vi "TLB Native Dynamic Events ver 0.26e.vi"() -> ()   [LabVIEW 2018] (continued)
                      shift-right: [w1907] -> w1904
                      shift-left: w1902 -> [w1906]
                      n658 = Enqueue Element(queue=w1906, element=w1905) -> (queue out=w1907:refnum<queue>)  [unwired: 2 in, 2 out]
                    }
                  }
                  frame True {
                    n659 = for {
                      shift-right: [w1912] -> w1910
                      shift-left: w1908 -> [w1913]
                      tunnel: string[] ["READ STEPPER VALUES", "", ""] -> [w1911] mode=indexing
                      n660 = Enqueue Element(queue=w1913, element=w1911) -> (queue out=w1912:refnum<queue>)  [unwired: 2 in, 2 out]
                    }
                  }
                }
                n661 = Or(x=w1895, y=w1891) -> (x .or. y?=w1898:bool)
                n662 = Select(t=State_Type_Definitions,_for_0.26g_versions_and_later_2."True Stop" ("Enum"), s=w1891, f=State_Type_Definitions,_for_0.26g_versions_and_later_2."Task 8K: RAISE MY SWORD" ("Enum")) -> (s? t:f=w1893:T18)
                n663 = Select(t=w1893, s=w1898, f=State_Type_Definitions,_for_0.26g_versions_and_later_2."Task 8J: CLOSE CLAW" ("Enum")) -> (s? t:f=w1897:T18)
              }
              frame "Exit" {
                n664 = for {
                  shift-right: [w1920] -> w1917
                  shift-left: w1914 -> [w1921]
                  tunnel: string[] ["STOP", "RESET ENCODERS", "RESET YAW", "ARDUINO MODE 0"] -> [w1919] mode=indexing
                  n665 = Enqueue Element(queue=w1921, element=w1919) -> (queue out=w1920:refnum<queue>)  [unwired: 2 in, 2 out]
                }
              }
            }
          }
          frame 37 {
            # ">>> yStepper command>>>"
            # ">> Manual override >>"
            n666 = Dequeue Element(queue=w1932, timeout in ms (-1)=w1931, error in (no error)=w1933) -> (element=w1930:T10)  [unwired: 3 out]
            n667 = Equal?(x=w1929, y=u8 60) -> (x = y?=w1927:bool)
            n668 = case shown="\"Start Task 1\", Default" w1930 {
              tunnel: [w1943 State_Type_Definitions,_for_0.26g_versions_and_later_2."True Stop" ("Enum")] -> w1934
              tunnel: [w1946 w1963] -> w1935
              tunnel: [State_Type_Definitions,_for_0.26g_versions_and_later_2."Idle" ("Enum") State_Type_Definitions,_for_0.26g_versions_and_later_2."Shutdown" ("Enum")] -> w1936
              tunnel: w1927 -> [w1942 _]
              tunnel: w1926 -> [w1941 _]
              tunnel: w1925 -> [w1937 w1960]
              frame "Start Task 1", Default {
                # "Stays in Task 5_A until stepper reaches desired \nheight"
                # "T: Go back to idle, F: Continue with task\""
                # ">> Manual override >>"
                n669 = case shown="True" w1942 {
                  tunnel: [w1950 w1956] -> w1946
                  tunnel: w1937 -> [w1948 w1954]
                  frame False {
                    n670 = for {
                      tunnel: string[] ["Z STEPPER CAM HEIGHT", "READ STEPPER VALUES"] ("element") -> [w1951] mode=indexing
                      shift-right: [w1953] -> w1950
                      shift-left: w1948 -> [w1952]
                      n671 = Enqueue Element(queue=w1952, element=w1951) -> (queue out=w1953:refnum<queue>)  [unwired: 2 in, 2 out]
                    }
                  }
                  frame True {
                    n672 = for {
                      shift-right: [w1958] -> w1956
                      shift-left: w1954 -> [w1959]
                      tunnel: string[] ["CAM CLOSE", "DISPOSE CAM BUFFERS", "DISPOSE PROC BUFFERS", "RESET ENCODERS"] -> [w1957] mode=indexing
                      n673 = Enqueue Element(queue=w1959, element=w1957) -> (queue out=w1958:refnum<queue>)  [unwired: 2 in, 2 out]
                    }
                  }
                }
                n674 = Or(x=w1942, y=w1941) -> (x .or. y?=w1944:bool)
                n675 = Select(t=State_Type_Definitions,_for_0.26g_versions_and_later_2."True Stop" ("Enum"), s=w1941, f=State_Type_Definitions,_for_0.26g_versions_and_later_2."True Stop" ("Enum")) -> (s? t:f=w1938:T18)
                n676 = Select(t=w1938, s=w1944, f=State_Type_Definitions,_for_0.26g_versions_and_later_2."Task 8K: RAISE MY SWORD" ("Enum")) -> (s? t:f=w1943:T18)
              }
              frame "Exit" {
                n677 = for {
                  shift-right: [w1966] -> w1963
                  shift-left: w1960 -> [w1967]
                  tunnel: string[] ["STOP", "RESET ENCODERS", "RESET YAW", "ARDUINO MODE 0"] -> [w1965] mode=indexing
                  n678 = Enqueue Element(queue=w1967, element=w1965) -> (queue out=w1966:refnum<queue>)  [unwired: 2 in, 2 out]
                }
              }
            }
          }
          frame 38 {
            # ">>> Motor control cluster >>>"
            # ">> Stepper height reeached >>"
            # ">>> yStepper command>>>"
            # ">> Manual override >>"
            n679 = Dequeue Element(queue=w1979, timeout in ms (-1)=w1974, error in (no error)=w1978) -> (element=w1982:T10)  [unwired: 3 out]
            n680 = Equal?(x=w1976, y=u8 50) -> (x = y?=w1980:bool)
            n681 = case shown="\"Start Task 1\", Default" w1982 {
              tunnel: [w1993 State_Type_Definitions,_for_0.26g_versions_and_later_2."True Stop" ("Enum")] -> w1972
              tunnel: [w1991 w2008] -> w1971
              tunnel: w1975 -> [w1990 _]
              tunnel: w1977 -> [w1984 _]
              tunnel: [State_Type_Definitions,_for_0.26g_versions_and_later_2."Idle" ("Enum") State_Type_Definitions,_for_0.26g_versions_and_later_2."Shutdown" ("Enum")] -> w1973
              tunnel: w1980 -> [w1983 _]
              frame "Start Task 1", Default {
                # ">> WIill proceed to part ii if not manual override >>"
                # ">>If ENABLE or Trigger is set to true>>"
                n682 = Or(x=w1983, y=w1984) -> (x .or. y?=w1985:bool)
                n683 = case shown="False" w1983 {
                  tunnel: [w1996 w2002] -> w1991
                  tunnel: w1990 -> [w1995 w2001]
                  frame False {
                    n684 = for {
                      shift-right: [w1998] -> w1996
                      shift-left: w1995 -> [w1999]
                      tunnel: string[] ["Z STEPPER BOX HEIGHT", "READ STEPPER VALUES"] ("element") -> [w1997] mode=indexing
                      n685 = Enqueue Element(queue=w1999, element=w1997) -> (queue out=w1998:refnum<queue>)  [unwired: 2 in, 2 out]
                    }
                  }
                  frame True {
                    n686 = for {
                      shift-right: [w2004] -> w2002
                      shift-left: w2001 -> [w2005]
                      tunnel: string[] ["READ NAVX", "RESET FLAGS", "RESET YAW", "", "", ""] -> [w2003] mode=indexing
                      n687 = Enqueue Element(queue=w2005, element=w2003) -> (queue out=w2004:refnum<queue>)  [unwired: 2 in, 2 out]
                    }
                  }
                }
                n688 = Select(t=State_Type_Definitions,_for_0.26g_versions_and_later_2."True Stop" ("Enum"), s=w1984, f=State_Type_Definitions,_for_0.26g_versions_and_later_2."Task 9B: Rotate to Angle" ("Enum")) -> (s? t:f=w1987:T18)
                n689 = Select(t=w1987, s=w1985, f=State_Type_Definitions,_for_0.26g_versions_and_later_2."Task 9A: Raise Arm" ("Enum")) -> (s? t:f=w1993:T18)
              }
              frame "Exit" {
                n690 = for {
                  shift-right: [w2011] -> w2008
                  shift-left: _ -> [w2012]
                  tunnel: string[] ["STOP", "RESET ENCODERS", "RESET YAW", ""] -> [w2010] mode=indexing
                  n691 = Enqueue Element(queue=w2012, element=w2010) -> (queue out=w2011:refnum<queue>)  [unwired: 2 in, 2 out]
                }
              }
            }
          }
          frame 39 {
            # ">>> Motor control cluster >>>"
            # ">>> yStepper command>>>"
            n692 = Dequeue Element(queue=w2026, timeout in ms (-1)=w2025, error in (no error)=w2024) -> (element=w2028:T10)  [unwired: 3 out]
            n693 = In Range and Coerce(upper limit=65.0, x=w2018, lower limit=58.0) -> (In Range?=w2015:bool)  [unwired: 1 out]
            n694 = case shown="\"Start Task 1\", Default" w2028 {
              tunnel: w2019 -> [w2031 _]
              tunnel: [w2039 State_Type_Definitions,_for_0.26g_versions_and_later_2."True Stop" ("Enum")] -> w2021
              tunnel: w2027 -> [w2037 w2055]
              tunnel: [w2036 w2054] -> w2020
              tunnel: [State_Type_Definitions,_for_0.26g_versions_and_later_2."Idle" ("Enum") State_Type_Definitions,_for_0.26g_versions_and_later_2."Shutdown" ("Enum")] -> w2022
              tunnel: w2015 -> [w2029 _]
              frame "Start Task 1", Default {
                n695 = Or(x=w2029, y=w2031) -> (x .or. y?=w2030:bool)
                n696 = case shown="False" w2029 {
                  tunnel: w2037 -> [w2042 w2048]
                  tunnel: [w2041 w2046] -> w2036
                  frame False {
                    n697 = for {
                      shift-right: [w2044] -> w2041
                      shift-left: w2042 -> [w2045]
                      tunnel: string[] ["READ NAVX", "R-CW", ""] ("element") -> [w2043] mode=indexing
                      n698 = Enqueue Element(queue=w2045, element=w2043) -> (queue out=w2044:refnum<queue>)  [unwired: 2 in, 2 out]
                    }
                  }
                  frame True {
                    n699 = for {
                      shift-right: [w2050] -> w2046
                      shift-left: w2048 -> [w2051]
                      tunnel: string[] ["STOP", "RESET ENCODERS", "RESET YAW", "", ""] -> [w2049] mode=indexing
                      n700 = Enqueue Element(queue=w2051, element=w2049) -> (queue out=w2050:refnum<queue>)  [unwired: 2 in, 2 out]
                    }
                  }
                }
                n701 = Select(t=State_Type_Definitions,_for_0.26g_versions_and_later_2."True Stop" ("Enum"), s=w2031, f=State_Type_Definitions,_for_0.26g_versions_and_later_2."Task 9C: Detect Box") -> (s? t:f=w2033:T18)
                n702 = Select(t=w2033, s=w2030, f=State_Type_Definitions,_for_0.26g_versions_and_later_2."Task 9B: Rotate to Angle" ("Enum")) -> (s? t:f=w2039:T18)
              }
              frame "Exit" {
                n703 = for {
                  shift-right: [w2058] -> w2054
                  shift-left: w2055 -> [w2059]
                  tunnel: string[] ["STOP", "RESET ENCODERS", "RESET YAW", ""] -> [w2057] mode=indexing
                  n704 = Enqueue Element(queue=w2059, element=w2057) -> (queue out=w2058:refnum<queue>)  [unwired: 2 in, 2 out]
                }
              }
            }
          }
          frame 40 {
            # ">>> Motor control cluster >>>"
            # ">>Line Detected>>"
            # ">>Action Queue>>"
            # ">>> yStepper command>>>"
            n705 = Dequeue Element(queue=w2071, timeout in ms (-1)=w2070, error in (no error)=w2069) -> (element=w2072:T10)  [unwired: 3 out]
            n706 = case shown="\"Start Task 1\", Default" w2072 {
              tunnel: w2067 -> [w2073 _]
              tunnel: [w2083 State_Type_Definitions,_for_0.26g_versions_and_later_2."True Stop" ("Enum")] -> w2064
              tunnel: w2068 -> [w2081 w2099]
              tunnel: [w2080 w2098] -> w2063
              tunnel: [State_Type_Definitions,_for_0.26g_versions_and_later_2."Idle" ("Enum") State_Type_Definitions,_for_0.26g_versions_and_later_2."Shutdown" ("Enum")] -> w2066
              tunnel: w2061 -> [w2074 _]
              frame "Start Task 1", Default {
                n707 = Or(x=w2073, y=w2074) -> (x .or. y?=w2075:bool)
                n708 = case shown="False" w2074 {
                  tunnel: w2081 -> [w2086 w2092]
                  tunnel: [w2085 w2090] -> w2080
                  frame False {
                    n709 = for {
                      shift-right: [w2088] -> w2085
                      shift-left: w2086 -> [w2089]
                      tunnel: string[] ["READ IR", "READ LINE SENSOR", "FORWARD - IR ASSIST"] ("element") -> [w2087] mode=indexing
                      n710 = Enqueue Element(queue=w2089, element=w2087) -> (queue out=w2088:refnum<queue>)  [unwired: 2 in, 2 out]
                    }
                  }
                  frame True {
                    n711 = for {
                      shift-right: [w2094] -> w2090
                      shift-left: w2092 -> [w2095]
                      tunnel: string[] ["STOP", "RESET ENCODERS", "RESET YAW", "RESET FLAGS"] -> [w2093] mode=indexing
                      n712 = Enqueue Element(queue=w2095, element=w2093) -> (queue out=w2094:refnum<queue>)  [unwired: 2 in, 2 out]
                    }
                  }
                }
                n713 = Select(t=State_Type_Definitions,_for_0.26g_versions_and_later_2."True Stop" ("Enum"), s=w2073, f=State_Type_Definitions,_for_0.26g_versions_and_later_2."Task 9D: MOVE FORWARD") -> (s? t:f=w2077:T18)
                n714 = Select(t=w2077, s=w2075, f=State_Type_Definitions,_for_0.26g_versions_and_later_2."Task 9C: Detect Box" ("Enum")) -> (s? t:f=w2083:T18)
              }
              frame "Exit" {
                n715 = for {
                  shift-right: [w2102] -> w2098
                  shift-left: w2099 -> [w2103]
                  tunnel: string[] ["STOP", "RESET ENCODERS", "RESET YAW", ""] -> [w2101] mode=indexing
                  n716 = Enqueue Element(queue=w2103, element=w2101) -> (queue out=w2102:refnum<queue>)  [unwired: 2 in, 2 out]
                }
              }
            }
          }
          frame 41 {
            (unwired) 50.0 ("y")
            # ">> Item Selection Bias >>"
            # ">> Wall detected >>"
            # ">> Manual override >>"
            # ">>Table Detected>>"
            # ">>> Motor control cluster >>>"
            # ">>Table or wall detectected>>"
            # ">>Action Queue>>"
            # ">>> yStepper command>>>"
            n717 = Dequeue Element(queue=w2121, timeout in ms (-1)=w2120, error in (no error)=w2119) -> (element=w2122:T10)  [unwired: 3 out]
            n718 = Less Or Equal?(x=w2110, y=18.0) -> (x <= y?=w2105:bool)
            n719 = Less?(x=w2108, y=20.0) -> (x < y?=w2106:bool)
            n720 = Or(x=w2105, y=w2106) -> (x .or. y?=w2104:bool)
            n721 = case shown="\"Start Task 1\", Default" w2122 {
              tunnel: w2117 -> [w2123 _]
              tunnel: [w2133 State_Type_Definitions,_for_0.26g_versions_and_later_2."True Stop" ("Enum")] -> w2114
              tunnel: w2118 -> [w2131 w2149]
              tunnel: [w2130 w2148] -> w2113
              tunnel: [State_Type_Definitions,_for_0.26g_versions_and_later_2."Idle" ("Enum") State_Type_Definitions,_for_0.26g_versions_and_later_2."Shutdown" ("Enum")] -> w2116
              tunnel: w2104 -> [w2124 _]
              frame "Start Task 1", Default {
                n722 = Or(x=w2123, y=w2124) -> (x .or. y?=w2125:bool)
                n723 = case shown="True" w2124 {
                  tunnel: w2131 -> [w2136 w2142]
                  tunnel: [w2135 w2140] -> w2130
                  frame False {
                    n724 = for {
                      shift-right: [w2138] -> w2135
                      shift-left: w2136 -> [w2139]
                      tunnel: string[] ["READ IR", "FORWARD - IR ASSIST", ""] ("element") -> [w2137] mode=indexing
                      n725 = Enqueue Element(queue=w2139, element=w2137) -> (queue out=w2138:refnum<queue>)  [unwired: 2 in, 2 out]
                    }
                  }
                  frame True {
                    n726 = for {
                      shift-right: [w2144] -> w2140
                      shift-left: w2142 -> [w2145]
                      tunnel: string[] ["STOP", "RESET ENCODERS", "RESET YAW", "RESET FLAGS"] -> [w2143] mode=indexing
                      n727 = Enqueue Element(queue=w2145, element=w2143) -> (queue out=w2144:refnum<queue>)  [unwired: 2 in, 2 out]
                    }
                  }
                }
                n728 = Select(t=State_Type_Definitions,_for_0.26g_versions_and_later_2."True Stop" ("Enum"), s=w2123, f=State_Type_Definitions,_for_0.26g_versions_and_later_2."Task 9E: MOVE LEFT") -> (s? t:f=w2127:T18)
                n729 = Select(t=w2127, s=w2125, f=State_Type_Definitions,_for_0.26g_versions_and_later_2."Task 9D: MOVE FORWARD" ("Enum")) -> (s? t:f=w2133:T18)
              }
              frame "Exit" {
                n730 = for {
                  shift-right: [w2152] -> w2148
                  shift-left: w2149 -> [w2153]
                  tunnel: string[] ["STOP", "RESET ENCODERS", "RESET YAW", ""] -> [w2151] mode=indexing
                  n731 = Enqueue Element(queue=w2153, element=w2151) -> (queue out=w2152:refnum<queue>)  [unwired: 2 in, 2 out]
                }
              }
            }
          }
          frame 42 {
            # ">> Item Selection Bias >>"
            # ">> Line detected? >>"
            # ">> Manual override >>"
            # ">>> Motor control cluster >>>"
            # ">>Action Queue>>"
            # ">>> yStepper command>>>"
            n732 = Dequeue Element(queue=w2165, timeout in ms (-1)=w2164, error in (no error)=w2163) -> (element=w2166:T10)  [unwired: 3 out]
            n733 = case shown="\"Start Task 1\", Default" w2166 {
              tunnel: w2161 -> [w2167 _]
              tunnel: [w2177 State_Type_Definitions,_for_0.26g_versions_and_later_2."True Stop" ("Enum")] -> w2158
              tunnel: w2162 -> [w2175 w2193]
              tunnel: [w2174 w2192] -> w2157
              tunnel: [State_Type_Definitions,_for_0.26g_versions_and_later_2."Idle" ("Enum") State_Type_Definitions,_for_0.26g_versions_and_later_2."Shutdown" ("Enum")] -> w2160
              tunnel: w2154 -> [w2168 _]
              frame "Start Task 1", Default {
                n734 = Or(x=w2167, y=w2168) -> (x .or. y?=w2169:bool)
                n735 = case shown="True" w2168 {
                  tunnel: w2175 -> [w2180 w2186]
                  tunnel: [w2179 w2184] -> w2174
                  frame False {
                    n736 = for {
                      shift-right: [w2182] -> w2179
                      shift-left: w2180 -> [w2183]
                      tunnel: string[] ["LEFT", "READ NAVX", "READ LINE SENSOR", ""] ("element") -> [w2181] mode=indexing
                      n737 = Enqueue Element(queue=w2183, element=w2181) -> (queue out=w2182:refnum<queue>)  [unwired: 2 in, 2 out]
                    }
                  }
                  frame True {
                    n738 = for {
                      shift-right: [w2188] -> w2184
                      shift-left: w2186 -> [w2189]
                      tunnel: string[] ["STOP", "RESET ENCODERS", "RESET YAW", "BOX COLOUR", "", ""] -> [w2187] mode=indexing
                      n739 = Enqueue Element(queue=w2189, element=w2187) -> (queue out=w2188:refnum<queue>)  [unwired: 2 in, 2 out]
                    }
                  }
                }
                n740 = Select(t=State_Type_Definitions,_for_0.26g_versions_and_later_2."True Stop" ("Enum"), s=w2167, f=State_Type_Definitions,_for_0.26g_versions_and_later_2."Task 9F: SCAN BOX") -> (s? t:f=w2171:T18)
                n741 = Select(t=w2171, s=w2169, f=State_Type_Definitions,_for_0.26g_versions_and_later_2."Task 9E: MOVE LEFT" ("Enum")) -> (s? t:f=w2177:T18)
              }
              frame "Exit" {
                n742 = for {
                  shift-right: [w2196] -> w2192
                  shift-left: w2193 -> [w2197]
                  tunnel: string[] ["STOP", "RESET ENCODERS", "RESET YAW", ""] -> [w2195] mode=indexing
                  n743 = Enqueue Element(queue=w2197, element=w2195) -> (queue out=w2196:refnum<queue>)  [unwired: 2 in, 2 out]
                }
              }
            }
          }
          frame 43 {
            # ">>> Motor control cluster >>>"
            # ">>Colour detection >>"
            # ">>> yStepper command>>>"
            # ">> Manual override >>"
            n744 = Dequeue Element(queue=w2214, timeout in ms (-1)=w2212, error in (no error)=w2213) -> (element=w2207:T10)  [unwired: 3 out]
            n745 = call "Box Colour FGV.vi"("Init/R/W State"=Box_Colour_FGV_States."Read") -> ("Colour to detect (output)"=w2199:T2)  [unwired: 9 in, 1 out]
            n746 = Equal?(x=w2200, y=w2199) -> (x = y?=w2198:bool)
            n747 = case shown="\"Start Task 1\", Default" w2207 {
              tunnel: [w2227 State_Type_Definitions,_for_0.26g_versions_and_later_2."True Stop" ("Enum")] -> w2203
              tunnel: [w2225 w2242] -> w2204
              tunnel: w2206 -> [w2224 _]
              tunnel: w2208 -> [w2217 _]
              tunnel: [State_Type_Definitions,_for_0.26g_versions_and_later_2."Idle" ("Enum") State_Type_Definitions,_for_0.26g_versions_and_later_2."Shutdown" ("Enum")] -> w2202
              tunnel: w2205 -> [w2218 _]
              tunnel: w2198 -> [w2216 _]
              frame "Start Task 1", Default {
                # ">> Will stop either due to manual override or is same box colour >>"
                # ">> WIill proceed to part ii if not manual override >>"
                # ">>If ENABLE or Trigger is set to true>>"
                n748 = Or(x=w2218, y=w2217) -> (x .or. y?=w2219:bool)
                n749 = case shown="True" w2218 {
                  tunnel: [w2230 w2236] -> w2225
                  tunnel: w2224 -> [w2229 w2235]
                  frame False {
                    n750 = for {
                      shift-right: [w2232] -> w2230
                      shift-left: w2229 -> [w2233]
                      tunnel: string[] ["", ""] ("element") -> [w2231] mode=indexing
                      n751 = Enqueue Element(queue=w2233, element=w2231) -> (queue out=w2232:refnum<queue>)  [unwired: 2 in, 2 out]
                    }
                  }
                  frame True {
                    n752 = for {
                      shift-right: [w2238] -> w2236
                      shift-left: w2235 -> [w2239]
                      tunnel: string[] ["RESET ENCODER", "RESET FLAGS", "RESET YAW", "", "", ""] -> [w2237] mode=indexing
                      n753 = Enqueue Element(queue=w2239, element=w2237) -> (queue out=w2238:refnum<queue>)  [unwired: 2 in, 2 out]
                    }
                  }
                }
                n754 = Or(x=w2217, y=w2216) -> (x .or. y?=w2215:bool)
                n755 = Select(t=State_Type_Definitions,_for_0.26g_versions_and_later_2."True Stop" ("Enum"), s=w2215, f=State_Type_Definitions,_for_0.26g_versions_and_later_2."Task 9G: MOVE RIGHT" ("Enum")) -> (s? t:f=w2221:T18)
                n756 = Select(t=w2221, s=w2219, f=State_Type_Definitions,_for_0.26g_versions_and_later_2."Task 9F: SCAN BOX" ("Enum")) -> (s? t:f=w2227:T18)
              }
              frame "Exit" {
                n757 = for {
                  shift-right: [w2245] -> w2242
                  shift-left: _ -> [w2246]
                  tunnel: string[] ["STOP", "RESET ENCODERS", "RESET YAW", ""] -> [w2244] mode=indexing
                  n758 = Enqueue Element(queue=w2246, element=w2244) -> (queue out=w2245:refnum<queue>)  [unwired: 2 in, 2 out]
                }
              }
            }
          }
          frame 44 {
            # ">>> Motor control cluster >>>"
            # ">>> yStepper command>>>"
            n759 = Dequeue Element(queue=w2258, timeout in ms (-1)=w2257, error in (no error)=w2256) -> (element=w2263:T10)  [unwired: 3 out]
            n760 = Greater?(x=w2248, y=50.0) -> (0:w2251:bool)
            n761 = And(x=w2249, y=w2251) -> (x .and. y?=w2247:bool)
            n762 = case shown="\"Start Task 1\", Default" w2263 {
              tunnel: w2247 -> [w2266 _]
              tunnel: [w2273 State_Type_Definitions,_for_0.26g_versions_and_later_2."True Stop" ("Enum")] -> w2262
              tunnel: w2255 -> [w2265 _]
              tunnel: w2259 -> [w2272 w2289]
              tunnel: [w2271 w2290] -> w2261
              tunnel: [State_Type_Definitions,_for_0.26g_versions_and_later_2."Idle" ("Enum") State_Type_Definitions,_for_0.26g_versions_and_later_2."Shutdown" ("Enum")] -> w2260
              frame "Start Task 1", Default {
                n763 = case shown="True" w2266 {
                  tunnel: w2272 -> [w2276 w2283]
                  tunnel: [w2277 w2282] -> w2271
                  frame False {
                    n764 = for {
                      tunnel: string[] ["READ LINE SENSOR", "READ NAVX", "RIGHT", "READ ENCODERS"] ("element") -> [w2278] mode=indexing
                      shift-right: [w2280] -> w2277
                      shift-left: w2276 -> [w2279]
                      n765 = Enqueue Element(queue=w2279, element=w2278) -> (queue out=w2280:refnum<queue>)  [unwired: 2 in, 2 out]
                    }
                  }
                  frame True {
                    n766 = for {
                      shift-right: [w2285] -> w2282
                      shift-left: w2283 -> [w2286]
                      tunnel: string[] ["RESET ENCODERS", "RESET YAW", "RESET FLAGS", "STOP", "BOX COLOUR"] -> [w2284] mode=indexing
                      n767 = Enqueue Element(queue=w2286, element=w2284) -> (queue out=w2285:refnum<queue>)  [unwired: 2 in, 2 out]
                    }
                  }
                }
                n768 = Or(x=w2266, y=w2265) -> (x .or. y?=w2264:bool)
                n769 = Select(t=State_Type_Definitions,_for_0.26g_versions_and_later_2."True Stop" ("Enum"), s=w2265, f=State_Type_Definitions,_for_0.26g_versions_and_later_2."Task 9H: SCAN BOX 2" ("Enum")) -> (s? t:f=w2267:T18)
                n770 = Select(t=w2267, s=w2264, f=State_Type_Definitions,_for_0.26g_versions_and_later_2."Task 9G: MOVE RIGHT" ("Enum")) -> (s? t:f=w2273:T18)
              }
              frame "Exit" {
                n771 = for {
                  shift-right: [w2293] -> w2290
                  shift-left: w2289 -> [w2294]
                  tunnel: string[] ["STOP", "RESET ENCODERS", "RESET YAW", "ARDUINO MODE 0"] -> [w2292] mode=indexing
                  n772 = Enqueue Element(queue=w2294, element=w2292) -> (queue out=w2293:refnum<queue>)  [unwired: 2 in, 2 out]
                }
              }
            }
          }
          frame 45 {
            # ">> Item Selection Bias >>"
            # ">>> Motor control cluster >>>"
            # ">>> yStepper command>>>"
            n773 = Dequeue Element(queue=w2304, timeout in ms (-1)=w2305, error in (no error)=w2306) -> (element=w2308:T10)  [unwired: 3 out]
            n774 = call "Box Colour FGV.vi"("Init/R/W State"=Box_Colour_FGV_States."Read") -> ("Colour to detect (output)"=w2297:T2)  [unwired: 9 in, 1 out]
            n775 = Equal?(x=w2296, y=w2297) -> (x = y?=w2295:bool)
            n776 = case shown="\"Start Task 1\", Default" w2308 {
              tunnel: w2299 -> [w2316 _]
              tunnel: [w2323 State_Type_Definitions,_for_0.26g_versions_and_later_2."True Stop" ("Enum")] -> w2301
              tunnel: w2307 -> [w2313 _]
              tunnel: w2303 -> [w2322 w2339]
              tunnel: [w2321 w2340] -> w2302
              tunnel: [State_Type_Definitions,_for_0.26g_versions_and_later_2."Idle" ("Enum") State_Type_Definitions,_for_0.26g_versions_and_later_2."Shutdown" ("Enum")] -> w2300
              tunnel: w2295 -> [w2314 _]
              frame "Start Task 1", Default {
                n777 = Or(x=w2316, y=w2313) -> (x .or. y?=w2315:bool)
                n778 = Or(x=w2314, y=w2313) -> (x .or. y?=w2312:bool)
                n779 = case shown="True" w2316 {
                  tunnel: w2322 -> [w2326 w2333]
                  tunnel: [w2327 w2332] -> w2321
                  frame False {
                    n780 = for {
                      tunnel: string[] ["", "", "", ""] ("element") -> [w2328] mode=indexing
                      shift-right: [w2330] -> w2327
                      shift-left: w2326 -> [w2329]
                      n781 = Enqueue Element(queue=w2329, element=w2328) -> (queue out=w2330:refnum<queue>)  [unwired: 2 in, 2 out]
                    }
                  }
                  frame True {
                    n782 = for {
                      shift-right: [w2335] -> w2332
                      shift-left: w2333 -> [w2336]
                      tunnel: string[] ["READ NAVX", "RESET FLAGS", "RESET ENCODERS", "", "", ""] -> [w2334] mode=indexing
                      n783 = Enqueue Element(queue=w2336, element=w2334) -> (queue out=w2335:refnum<queue>)  [unwired: 2 in, 2 out]
                    }
                  }
                }
                n784 = Select(t=State_Type_Definitions,_for_0.26g_versions_and_later_2."True Stop" ("Enum"), s=w2312, f=State_Type_Definitions,_for_0.26g_versions_and_later_2."Task 9I: ROTATE 90 CW" ("Enum")) -> (s? t:f=w2317:T18)
                n785 = Select(t=w2317, s=w2315, f=State_Type_Definitions,_for_0.26g_versions_and_later_2."Task 9H: SCAN BOX 2" ("Enum")) -> (s? t:f=w2323:T18)
              }
              frame "Exit" {
                n786 = for {
                  shift-right: [w2343] -> w2340
                  shift-left: w2339 -> [w2344]
                  tunnel: string[] ["STOP", "RESET ENCODERS", "RESET YAW", "ARDUINO MODE 0"] -> [w2342] mode=indexing
                  n787 = Enqueue Element(queue=w2344, element=w2342) -> (queue out=w2343:refnum<queue>)  [unwired: 2 in, 2 out]
                }
              }
            }
          }
          frame 46 {
            # ">> Item Selection Bias >>"
            n788 = Dequeue Element(queue=w2348, timeout in ms (-1)=w2349, error in (no error)=w2350) -> (element=w2356:T10)  [unwired: 3 out]
            n789 = Less?(x=w2346, y=-38.0) -> (x < y?=w2345:bool)
            n790 = case shown="\"Start Task 1\", Default" w2356 {
              tunnel: w2345 -> [w2362 _]
              tunnel: [w2369 State_Type_Definitions,_for_0.26g_versions_and_later_2."True Stop" ("Enum")] -> w2353
              tunnel: w2351 -> [w2361 _]
              tunnel: w2355 -> [w2368 w2385]
              tunnel: [w2367 w2386] -> w2354
              tunnel: [State_Type_Definitions,_for_0.26g_versions_and_later_2."Idle" ("Enum") State_Type_Definitions,_for_0.26g_versions_and_later_2."Shutdown" ("Enum")] -> w2352
              frame "Start Task 1", Default {
                n791 = case shown="False" w2362 {
                  tunnel: w2368 -> [w2372 w2379]
                  tunnel: [w2373 w2378] -> w2367
                  frame False {
                    n792 = for {
                      tunnel: string[] ["R-CW", "READ ENCODERS", ""] ("element") -> [w2374] mode=indexing
                      shift-right: [w2376] -> w2373
                      shift-left: w2372 -> [w2375]
                      n793 = Enqueue Element(queue=w2375, element=w2374) -> (queue out=w2376:refnum<queue>)  [unwired: 2 in, 2 out]
                    }
                  }
                  frame True {
                    n794 = for {
                      shift-right: [w2381] -> w2378
                      shift-left: w2379 -> [w2382]
                      tunnel: string[] ["STOP", "RESET ENCODERS", "RESET YAW", "RESET FLAGS", "", ""] -> [w2380] mode=indexing
                      n795 = Enqueue Element(queue=w2382, element=w2380) -> (queue out=w2381:refnum<queue>)  [unwired: 2 in, 2 out]
                    }
                  }
                }
                n796 = Or(x=w2362, y=w2361) -> (x .or. y?=w2360:bool)
                n797 = Select(t=State_Type_Definitions,_for_0.26g_versions_and_later_2."True Stop" ("Enum"), s=w2361, f=State_Type_Definitions,_for_0.26g_versions_and_later_2."Task 9J: FORWARD" ("Enum")) -> (s? t:f=w2363:T18)
                n798 = Select(t=w2363, s=w2360, f=State_Type_Definitions,_for_0.26g_versions_and_later_2."Task 9I: ROTATE 90 CW" ("Enum")) -> (s? t:f=w2369:T18)
              }
              frame "Exit" {
                n799 = for {
                  shift-right: [w2389] -> w2386
                  shift-left: w2385 -> [w2390]
                  tunnel: string[] ["STOP", "RESET ENCODERS", "RESET YAW", "ARDUINO MODE 0"] -> [w2388] mode=indexing
                  n800 = Enqueue Element(queue=w2390, element=w2388) -> (queue out=w2389:refnum<queue>)  [unwired: 2 in, 2 out]
                }
              }
            }
          }
          frame 47 {
            # ">>Stops if either table or wall is obstructing >>"
            # ">> Item Selection Bias >>"
            n801 = Less?(x=w2395, y=50.0) -> (x < y?=w2394:bool)
            n802 = Less?(x=w2398, y=20.0) -> (x < y?=w2396:bool)
            n803 = Not Equal To 0?(x=w2395) -> (x != 0?=w2393:bool)
            n804 = Not Equal To 0?(x=w2398) -> (x != 0?=w2397:bool)
            n805 = And(x=w2393, y=w2394) -> (x .and. y?=w2391:bool)
            n806 = And(x=w2397, y=w2396) -> (x .and. y?=w2392:bool)
            n807 = Dequeue Element(queue=w2406, timeout in ms (-1)=w2407, error in (no error)=w2408) -> (element=w2410:T10)  [unwired: 3 out]
            n808 = Or(x=w2392, y=w2391) -> (x .or. y?=w2399:bool)
            n809 = case shown="\"Start Task 1\", Default" w2410 {
              tunnel: w2399 -> [w2416 _]
              tunnel: [w2423 State_Type_Definitions,_for_0.26g_versions_and_later_2."True Stop" ("Enum")] -> w2404
              tunnel: w2409 -> [w2415 _]
              tunnel: w2405 -> [w2422 w2439]
              tunnel: [w2421 w2440] -> w2403
              tunnel: [State_Type_Definitions,_for_0.26g_versions_and_later_2."Idle" ("Enum") State_Type_Definitions,_for_0.26g_versions_and_later_2."Shutdown" ("Enum")] -> w2402
              frame "Start Task 1", Default {
                n810 = case shown="False" w2416 {
                  tunnel: w2422 -> [w2426 w2433]
                  tunnel: [w2427 w2432] -> w2421
                  frame False {
                    n811 = for {
                      tunnel: string[] ["READ IR", "READ NAVX", "FORWARD"] ("element") -> [w2428] mode=indexing
                      shift-right: [w2430] -> w2427
                      shift-left: w2426 -> [w2429]
                      n812 = Enqueue Element(queue=w2429, element=w2428) -> (queue out=w2430:refnum<queue>)  [unwired: 2 in, 2 out]
                    }
                  }
                  frame True {
                    n813 = for {
                      shift-right: [w2435] -> w2432
                      shift-left: w2433 -> [w2436]
                      tunnel: string[] ["STOP", "RESET ENCODERS", "RESET YAW", "RESET FLAGS", "", ""] -> [w2434] mode=indexing
                      n814 = Enqueue Element(queue=w2436, element=w2434) -> (queue out=w2435:refnum<queue>)  [unwired: 2 in, 2 out]
                    }
                  }
                }
                n815 = Or(x=w2416, y=w2415) -> (x .or. y?=w2414:bool)
                n816 = Select(t=State_Type_Definitions,_for_0.26g_versions_and_later_2."True Stop" ("Enum"), s=w2415, f=State_Type_Definitions,_for_0.26g_versions_and_later_2."True Stop" ("Enum")) -> (s? t:f=w2417:T18)
                n817 = Select(t=w2417, s=w2414, f=State_Type_Definitions,_for_0.26g_versions_and_later_2."Task 9J: FORWARD" ("Enum")) -> (s? t:f=w2423:T18)
              }
              frame "Exit" {
                n818 = for {
                  shift-right: [w2443] -> w2440
                  shift-left: w2439 -> [w2444]
                  tunnel: string[] ["STOP", "RESET ENCODERS", "RESET YAW", "ARDUINO MODE 0"] -> [w2442] mode=indexing
                  n819 = Enqueue Element(queue=w2444, element=w2442) -> (queue out=w2443:refnum<queue>)  [unwired: 2 in, 2 out]
                }
              }
            }
          }
          frame 48 {
            # ">>> Motor control cluster >>>"
            # ">>> yStepper command>>>"
            # ">> Item Selection Bias >>"
            n820 = Less?(x=w2448, y=-38.0) -> (x < y?=w2446:bool)
            n821 = Dequeue Element(queue=w2454, timeout in ms (-1)=w2453, error in (no error)=w2452) -> (element=w2456:T10)  [unwired: 3 out]
            n822 = case shown="\"Start Task 1\", Default" w2456 {
              tunnel: w2446 -> [w2462 _]
              tunnel: [w2469 State_Type_Definitions,_for_0.26g_versions_and_later_2."True Stop" ("Enum")] -> w2450
              tunnel: w2451 -> [w2461 _]
              tunnel: w2455 -> [w2468 w2485]
              tunnel: [w2467 w2486] -> w2445
              tunnel: [State_Type_Definitions,_for_0.26g_versions_and_later_2."Idle" ("Enum") State_Type_Definitions,_for_0.26g_versions_and_later_2."Shutdown" ("Enum")] -> w2449
              frame "Start Task 1", Default {
                n823 = case shown="True" w2462 {
                  tunnel: w2468 -> [w2472 w2479]
                  tunnel: [w2473 w2478] -> w2467
                  frame False {
                    n824 = for {
                      tunnel: string[] ["READ ENCODERS", "R-CW"] ("element") -> [w2474] mode=indexing
                      shift-right: [w2476] -> w2473
                      shift-left: w2472 -> [w2475]
                      n825 = Enqueue Element(queue=w2475, element=w2474) -> (queue out=w2476:refnum<queue>)  [unwired: 2 in, 2 out]
                    }
                  }
                  frame True {
                    n826 = for {
                      shift-right: [w2481] -> w2478
                      shift-left: w2479 -> [w2482]
                      tunnel: string[] ["STOP", "RESET ENCODERS", "RESET FLAGS", "RESET YAW", "READ IR", "ARDUINO - ULTRASONIC"] -> [w2480] mode=indexing
                      n827 = Enqueue Element(queue=w2482, element=w2480) -> (queue out=w2481:refnum<queue>)  [unwired: 2 in, 2 out]
                    }
                  }
                }
                n828 = Or(x=w2462, y=w2461) -> (x .or. y?=w2460:bool)
                n829 = Select(t=State_Type_Definitions,_for_0.26g_versions_and_later_2."True Stop" ("Enum"), s=w2461, f=State_Type_Definitions,_for_0.26g_versions_and_later_2."Task 9L: SCAN BOX 3" ("Enum")) -> (s? t:f=w2463:u16)
                n830 = Select(t=w2463, s=w2460, f=State_Type_Definitions,_for_0.26g_versions_and_later_2."Task 9K: MOVE RIGHT" ("Enum")) -> (s? t:f=w2469:u16)
              }
              frame "Exit" {
                n831 = for {
                  shift-right: [w2489] -> w2486
                  shift-left: w2485 -> [w2490]
                  tunnel: string[] ["STOP", "RESET ENCODERS", "RESET YAW", "ARDUINO MODE 0"] -> [w2488] mode=indexing
                  n832 = Enqueue Element(queue=w2490, element=w2488) -> (queue out=w2489:refnum<queue>)  [unwired: 2 in, 2 out]
                }
              }
            }
          }
          frame 49 {
            w2503 = u8 50 ("y")
            # ">>> Motor control cluster >>>"
            # ">>> yStepper command>>>"
            # ">> Item Selection Bias >>"
            n833 = Less?(x=w2505, y=w2503) -> (x < y?=w2498:bool)
            n834 = Dequeue Element(queue=w2509, timeout in ms (-1)=w2508, error in (no error)=w2507) -> (element=w2513:T10)  [unwired: 3 out]
            n835 = Less?(x=w2504, y=w2503) -> (x < y?=w2499:bool)
            n836 = And(x=w2499, y=w2498) -> (x .and. y?=w2491:bool)
            n837 = Less Or Equal?(x=w2502, y=15.0) -> (x <= y?=w2497:bool)
            n838 = Greater?(x=w2496, y=100.0) -> (0:w2495:bool)
            n839 = Or(x=w2497, y=w2491) -> (x .or. y?=w2493:bool)
            n840 = And(x=w2495, y=w2493) -> (x .and. y?=w2494:bool)
            n841 = case shown="\"Start Task 1\", Default" w2513 {
              tunnel: w2494 -> [w2519 _]
              tunnel: [w2526 State_Type_Definitions,_for_0.26g_versions_and_later_2."True Stop" ("Enum")] -> w2511
              tunnel: w2506 -> [w2518 _]
              tunnel: w2510 -> [w2525 w2542]
              tunnel: [w2524 w2543] -> w2500
              tunnel: [State_Type_Definitions,_for_0.26g_versions_and_later_2."Idle" ("Enum") State_Type_Definitions,_for_0.26g_versions_and_later_2."Shutdown" ("Enum")] -> w2512
              frame "Start Task 1", Default {
                n842 = case shown="True" w2519 {
                  tunnel: w2525 -> [w2529 w2536]
                  tunnel: [w2530 w2535] -> w2524
                  frame False {
                    n843 = for {
                      tunnel: string[] ["READ IR", "FORWARD", "READ NAVX", "READ ENCODERS"] ("element") -> [w2531] mode=indexing
                      shift-right: [w2533] -> w2530
                      shift-left: w2529 -> [w2532]
                      n844 = Enqueue Element(queue=w2532, element=w2531) -> (queue out=w2533:refnum<queue>)  [unwired: 2 in, 2 out]
                    }
                  }
                  frame True {
                    n845 = for {
                      shift-right: [w2538] -> w2535
                      shift-left: w2536 -> [w2539]
                      tunnel: string[] ["STOP", "RESET ENCODERS", "RESET FLAGS", "RESET YAW", "", ""] -> [w2537] mode=indexing
                      n846 = Enqueue Element(queue=w2539, element=w2537) -> (queue out=w2538:refnum<queue>)  [unwired: 2 in, 2 out]
                    }
                  }
                }
                n847 = Or(x=w2519, y=w2518) -> (x .or. y?=w2517:bool)
                n848 = Select(t=State_Type_Definitions,_for_0.26g_versions_and_later_2."True Stop" ("Enum"), s=w2518, f=State_Type_Definitions,_for_0.26g_versions_and_later_2."True Stop" ("Enum")) -> (s? t:f=w2520:T18)
                n849 = Select(t=w2520, s=w2517, f=State_Type_Definitions,_for_0.26g_versions_and_later_2."Task 9L: SCAN BOX 3" ("Enum")) -> (s? t:f=w2526:u16)
              }
              frame "Exit" {
                n850 = for {
                  shift-right: [w2546] -> w2543
                  shift-left: w2542 -> [w2547]
                  tunnel: string[] ["STOP", "RESET ENCODERS", "RESET YAW", "ARDUINO MODE 0"] -> [w2545] mode=indexing
                  n851 = Enqueue Element(queue=w2547, element=w2545) -> (queue out=w2546:refnum<queue>)  [unwired: 2 in, 2 out]
                }
              }
            }
          }
          frame 51 {
            # ">> Item Selection Bias >>"
            n852 = Dequeue Element(queue=w2552, timeout in ms (-1)=w2551, error in (no error)=w2550) -> (element=w2557:T10)  [unwired: 3 out]
            n853 = case shown="\"Start Task 1\", Default" w2557 {
              tunnel: w2548 -> [w2563 _]
              tunnel: [w2570 State_Type_Definitions,_for_0.26g_versions_and_later_2."True Stop" ("Enum")] -> w2555
              tunnel: w2549 -> [w2562 _]
              tunnel: w2553 -> [w2569 w2586]
              tunnel: [w2568 w2587] -> w2554
              tunnel: [State_Type_Definitions,_for_0.26g_versions_and_later_2."Idle" ("Enum") State_Type_Definitions,_for_0.26g_versions_and_later_2."Shutdown" ("Enum")] -> w2556
              frame "Start Task 1", Default {
                n854 = case shown="False" w2563 {
                  tunnel: w2569 -> [w2573 w2580]
                  tunnel: [w2574 w2579] -> w2568
                  frame False {
                    n855 = for {
                      tunnel: string[] ["READ LINE SENSOR", "READ NAVX", "RIGHT", "READ ENCODERS"] ("element") -> [w2575] mode=indexing
                      shift-right: [w2577] -> w2574
                      shift-left: w2573 -> [w2576]
                      n856 = Enqueue Element(queue=w2576, element=w2575) -> (queue out=w2577:refnum<queue>)  [unwired: 2 in, 2 out]
                    }
                  }
                  frame True {
                    n857 = for {
                      shift-right: [w2582] -> w2579
                      shift-left: w2580 -> [w2583]
                      tunnel: string[] ["STOP", "RESET ENCODERS", "RESET YAW", "OPEN LIFE CAM", "SET TIMER 2", "RESET FLAGS"] -> [w2581] mode=indexing
                      n858 = Enqueue Element(queue=w2583, element=w2581) -> (queue out=w2582:refnum<queue>)  [unwired: 2 in, 2 out]
                    }
                  }
                }
                n859 = Or(x=w2563, y=w2562) -> (x .or. y?=w2561:bool)
                n860 = Select(t=State_Type_Definitions,_for_0.26g_versions_and_later_2."True Stop" ("Enum"), s=w2562, f=State_Type_Definitions,_for_0.26g_versions_and_later_2."Task 9N: SCAN BOX 4" ("Enum")) -> (s? t:f=w2564:T18)
                n861 = Select(t=w2564, s=w2561, f=State_Type_Definitions,_for_0.26g_versions_and_later_2."Task 9M: MOVE RIGHT" ("Enum")) -> (s? t:f=w2570:T18)
              }
              frame "Exit" {
                n862 = for {
                  shift-right: [w2590] -> w2587
                  shift-left: w2586 -> [w2591]
                  tunnel: string[] ["STOP", "RESET ENCODERS", "RESET YAW", "ARDUINO MODE 0"] -> [w2589] mode=indexing
                  n863 = Enqueue Element(queue=w2591, element=w2589) -> (queue out=w2590:refnum<queue>)  [unwired: 2 in, 2 out]
                }
              }
            }
          }
          frame 52 {
            # ">> Manual override >>"
            n864 = Dequeue Element(queue=w2600, timeout in ms (-1)=w2599, error in (no error)=w2598) -> (element=w2601:T10)  [unwired: 3 out]
            n865 = case shown="\"Start Task 1\", Default" w2601 {
              tunnel: [w2615 State_Type_Definitions,_for_0.26g_versions_and_later_2."True Stop" ("Enum")] -> w2593
              tunnel: [w2613 w2631] -> w2592
              tunnel: w2596 -> [w2612 w2628]
              tunnel: w2597 -> [w2606 _]
              tunnel: [State_Type_Definitions,_for_0.26g_versions_and_later_2."Idle" ("Enum") State_Type_Definitions,_for_0.26g_versions_and_later_2."Shutdown" ("Enum")] -> w2594
              tunnel: w2595 -> [w2605 _]
              frame "Start Task 1", Default {
                # ">> WIill proceed to part ii if not manual override >>"
                # ">>If ENABLE or Trigger is set to true>>"
                n866 = Or(x=w2605, y=w2606) -> (x .or. y?=w2607:bool)
                n867 = case shown="False" w2605 {
                  tunnel: [w2618 w2624] -> w2613
                  tunnel: w2612 -> [w2617 w2623]
                  frame False {
                    n868 = for {
                      shift-right: [w2620] -> w2618
                      shift-left: w2617 -> [w2621]
                      tunnel: string[] ["CAM ACQ", "START TIMER"] ("element") -> [w2619] mode=indexing
                      n869 = Enqueue Element(queue=w2621, element=w2619) -> (queue out=w2620:refnum<queue>)  [unwired: 2 in, 2 out]
                    }
                  }
                  frame True {
                    n870 = for {
                      shift-right: [w2626] -> w2624
                      shift-left: w2623 -> [w2627]
                      tunnel: string[] ["CLOSE CAM", "SET TIMER 5", "", "", "", ""] -> [w2625] mode=indexing
                      n871 = Enqueue Element(queue=w2627, element=w2625) -> (queue out=w2626:refnum<queue>)  [unwired: 2 in, 2 out]
                    }
                  }
                }
                n872 = Select(t=State_Type_Definitions,_for_0.26g_versions_and_later_2."True Stop" ("Enum"), s=w2606, f=State_Type_Definitions,_for_0.26g_versions_and_later_2."PENIS" ("Enum")) -> (s? t:f=w2609:T18)
                n873 = Select(t=w2609, s=w2607, f=State_Type_Definitions,_for_0.26g_versions_and_later_2."Task 9N: SCAN BOX 4" ("Enum")) -> (s? t:f=w2615:T18)
              }
              frame "Exit" {
                n874 = for {
                  shift-right: [w2634] -> w2631
                  shift-left: w2628 -> [w2635]
                  tunnel: string[] ["STOP", "RESET ENCODERS", "RESET YAW", ""] -> [w2633] mode=indexing
                  n875 = Enqueue Element(queue=w2635, element=w2633) -> (queue out=w2634:refnum<queue>)  [unwired: 2 in, 2 out]
                }
              }
            }
          }
          frame 53 {
            # ">> Item Selection Bias >>"
            n876 = Dequeue Element(queue=w2643, timeout in ms (-1)=w2642, error in (no error)=w2641) -> (element=w2645:T10)  [unwired: 3 out]
            n877 = case shown="\"Start Task 1\", Default" w2645 {
              tunnel: w2636 -> [w2651 _]
              tunnel: [w2658 State_Type_Definitions,_for_0.26g_versions_and_later_2."True Stop" ("Enum")] -> w2639
              tunnel: w2640 -> [w2650 _]
              tunnel: w2644 -> [w2657 w2674]
              tunnel: [w2656 w2675] -> w2638
              tunnel: [State_Type_Definitions,_for_0.26g_versions_and_later_2."Idle" ("Enum") State_Type_Definitions,_for_0.26g_versions_and_later_2."Shutdown" ("Enum")] -> w2637
              frame "Start Task 1", Default {
                n878 = case shown="False" w2651 {
                  tunnel: w2657 -> [w2661 w2668]
                  tunnel: [w2662 w2667] -> w2656
                  frame False {
                    n879 = for {
                      tunnel: string[] ["START TIMER", "COLOUR PROCESSING", ""] ("element") -> [w2663] mode=indexing
                      shift-right: [w2665] -> w2662
                      shift-left: w2661 -> [w2664]
                      n880 = Enqueue Element(queue=w2664, element=w2663) -> (queue out=w2665:refnum<queue>)  [unwired: 2 in, 2 out]
                    }
                  }
                  frame True {
                    n881 = for {
                      shift-right: [w2670] -> w2667
                      shift-left: w2668 -> [w2671]
                      tunnel: string[] ["CLOSE CAM", "DISPOSE BUFFERS", "RESET ENCODERS", "RESET YAW", "RESET FLAGS", ""] -> [w2669] mode=indexing
                      n882 = Enqueue Element(queue=w2671, element=w2669) -> (queue out=w2670:refnum<queue>)  [unwired: 2 in, 2 out]
                    }
                  }
                }
                n883 = Or(x=w2651, y=w2650) -> (x .or. y?=w2649:bool)
                n884 = Select(t=State_Type_Definitions,_for_0.26g_versions_and_later_2."True Stop" ("Enum"), s=w2650, f=State_Type_Definitions,_for_0.26g_versions_and_later_2."PENIS 2" ("Enum")) -> (s? t:f=w2652:T18)
                n885 = Select(t=w2652, s=w2649, f=State_Type_Definitions,_for_0.26g_versions_and_later_2."PENIS" ("Enum")) -> (s? t:f=w2658:T18)
              }
              frame "Exit" {
                n886 = for {
                  shift-right: [w2678] -> w2675
                  shift-left: w2674 -> [w2679]
                  tunnel: string[] ["STOP", "RESET ENCODERS", "RESET YAW", "ARDUINO MODE 0"] -> [w2677] mode=indexing
                  n887 = Enqueue Element(queue=w2679, element=w2677) -> (queue out=w2678:refnum<queue>)  [unwired: 2 in, 2 out]
                }
              }
            }
          }
          frame 54 {
            # ">> Item Selection Bias >>"
            n888 = Dequeue Element(queue=w2685, timeout in ms (-1)=w2684, error in (no error)=w2683) -> (element=w2693:T10)  [unwired: 3 out]
            n889 = Greater?(x=w2681, y=50.0) -> (0:w2691:bool)
            n890 = And(x=w2680, y=w2691) -> (x .and. y?=w2692:bool)
            n891 = case shown="\"Start Task 1\", Default" w2693 {
              tunnel: w2692 -> [w2699 _]
              tunnel: [w2706 State_Type_Definitions,_for_0.26g_versions_and_later_2."True Stop" ("Enum")] -> w2688
              tunnel: w2682 -> [w2698 _]
              tunnel: w2686 -> [w2705 w2722]
              tunnel: [w2704 w2723] -> w2687
              tunnel: [State_Type_Definitions,_for_0.26g_versions_and_later_2."Idle" ("Enum") State_Type_Definitions,_for_0.26g_versions_and_later_2."Shutdown" ("Enum")] -> w2689
              frame "Start Task 1", Default {
                n892 = case shown="False" w2699 {
                  tunnel: w2705 -> [w2709 w2716]